vi "UHR-Fleezers Control (host) - 12.8.vi"() -> ()   [LabVIEW 2012] (continued)
        n423 = flat-sequence {
          tunnel: w684 -> [w688]
          tunnel: w685 -> [w689]
          tunnel: [w689] -> w681
          tunnel: [w688] -> w680
          tunnel: w681 -> [w694]
          tunnel: w680 -> [w693]
          tunnel: ["Cal @ (MHz)"] -> w678
          tunnel: [w698] -> w682
          tunnel: w678 -> [w698]
          tunnel: w682 -> [w707]
          tunnel: ["W/ Offset 1"] -> w679
          tunnel: w682 -> [w728]
          tunnel: w679 -> [w726]
          frame #0 {
            n424 = property on="Sample Channel\nFlow" class="Bool (strict)"("Val(Sgnl)"="Daq spot flow on") -> ()  [unwired: 2 in, 2 out]
            n425 = Wait (ms)(milliseconds to wait=u32 250) -> ()  [unwired: 1 out]
          }
          frame #1 {
            n426 = local read "Saved Stage Positions"() -> (w691:dbl[][])
            n427 = property on="Trap Delta (MHz)" class="DigNum (strict)"("Val(Sgnl)"="Cal @ (MHz)") -> ()  [unwired: 2 in, 2 out]
            n428 = local write "Stage Moving"(TRUE ("Stage Moving")) -> ()
            n429 = call "move to saved stage position.vi"("error in"=w693, "Stage VISA resource name in"=w694, "Position"="Cal Stage Position", "Saved Stage Positions"=w691) -> ("error out"=w692:errorcluster)  [unwired: 1 out]
            n430 = local write "Stage Control Serial Error"(w692) -> ()
          }
          frame #2 {
            n431 = local write "Stage Moving"(FALSE ("Stage Moving")) -> ()
            n432 = property on="Sample Channel\nFlow" class="Bool (strict)"("Val(Sgnl)"="Flow ON during cal?") -> ()  [unwired: 2 in, 2 out]
            n433 = call <vilib>:"Beep.vi"() -> ()  [unwired: 3 in, 9 out]
          }
          frame #3 {
            n434 = Wait (ms)(milliseconds to wait=u32 1000) -> ()  [unwired: 1 out]
          }
          frame #4 {
            n435 = property on="Save Calibration" class="Bool (strict)"("Val(Sgnl)"=TRUE ("Value (Signaling)")) -> ()  [unwired: 2 in, 2 out]
          }
          frame #5 {
            n436 = Wait (ms)(milliseconds to wait=u32 2000) -> ()  [unwired: 1 out]
          }
          frame #6 {
            # "Check to see if \nsaving done"
            n437 = while {
              stop <- w703 stop-if-true
              n438 = local read "Saving..."() -> (w704:bool)
              n439 = Wait (ms)(milliseconds to wait=u32 100) -> ()  [unwired: 1 out]
              n440 = Not(x=w704) -> (.not. x?=w703:bool)
            }
          }
          frame #7 {
            n441 = case shown="True" "W/ Offset 1" {
              tunnel: w707 -> [_ w708]
              frame False {
              }
              frame True {
                n442 = stacked-sequence {
                  tunnel: w708 -> [_ _ _ _ _ _ _ w725]
                  frame #0 {
                    n443 = property on="Trap Delta (MHz)" class="DigNum (strict)"("Val(Sgnl)"="Offset 1 Start (MHz)") -> ()  [unwired: 2 in, 2 out]
                    n444 = Replace Array Subset(array=u32[] [0] ("Index Values"), new element="Offset 1 Set", index=0) -> (w709:u32[])
                    n445 = property on="Saved AOD Raster Scan Parameter Sets" class="Arr (strict)"("Index Values"=w709) -> ()  [unwired: 2 in, 2 out]
                  }
                  frame #1 {
                    n446 = Wait (ms)(milliseconds to wait=u32 200) -> ()  [unwired: 1 out]
                  }
                  frame #2 {
                    n447 = property on="Load parameters" class="Bool (strict)"("Val(Sgnl)"=TRUE ("Value (Signaling)")) -> ()  [unwired: 2 in, 2 out]
                  }
                  frame #3 {
                    n448 = Wait (ms)(milliseconds to wait=u32 200) -> ()  [unwired: 1 out]
                  }
                  frame #4 {
                    n449 = property on="Trap Raster Scan" class="Bool (strict)"("Val(Sgnl)"=TRUE ("Value (Signaling)")) -> ()  [unwired: 2 in, 2 out]
                  }
                  frame #5 {
                    n450 = Wait (ms)(milliseconds to wait=u32 2000) -> ()  [unwired: 1 out]
                  }
                  frame #6 {
                    n451 = while {
                      stop <- w722 stop-if-true
                      n452 = local read "Raster Scanning..."() -> (w724:bool)
                      n453 = local read "Saving..."() -> (w720:bool)
                      n454 = Wait (ms)(milliseconds to wait=u32 100) -> ()  [unwired: 1 out]
                      n455 = Not(x=w720) -> (.not. x?=w719:bool)
                      n456 = Not(x=w724) -> (.not. x?=w721:bool)
                      n457 = And(x=w721, y=w719) -> (x .and. y?=w722:bool)
                    }
                  }
                  frame #7 {
                    n458 = property on="Trap Delta (MHz)" class="DigNum (strict)"("Val(Sgnl)"=w725) -> ()  [unwired: 2 in, 2 out]
                  }
                }
              }
            }
          }
          frame #8 {
            n459 = local read "Save ave N"() -> (w727:dbl)
            n460 = case shown="False" "W/ Offset 2" {
              tunnel: w728 -> [_ w735]
              tunnel: w727 -> [_ w734]
              tunnel: w726 -> [w730 _]
              frame False {
                n461 = case shown="False" w730 {
                  frame False {
                    n462 = Multiply(x="Cal read wait (s)", y=u32 1000 ("milliseconds to wait")) -> (x*y=w732:u32)
                    n463 = Wait (ms)(milliseconds to wait=w732) -> ()  [unwired: 1 out]
                  }
                  frame True {
                  }
                }
              }
              frame True {
                n464 = stacked-sequence {
                  tunnel: w735 -> [_ _ _ _ _ _ _ _ _ w756 _ _]
                  tunnel: w734 -> [_ _ _ _ _ _ _ _ _ w754 _ _]
                  frame #0 {
                    n465 = property on="Save ave N" class="DigNum (strict)"("Val(Sgnl)"=1.0 ("Value (Signaling)")) -> ()  [unwired: 2 in, 2 out]
                  }
                  frame #1 {
                    n466 = Wait (ms)(milliseconds to wait=u32 500) -> ()  [unwired: 1 out]
                  }
                  frame #2 {
                    n467 = property on="Trap Delta (MHz)" class="DigNum (strict)"("Val(Sgnl)"="Offset 2 Start (MHz)") -> ()  [unwired: 2 in, 2 out]
                    n468 = Replace Array Subset(array=u32[] [0] ("Index Values"), new element="Offset 2 Set", index=0) -> (w740:u32[])
                    n469 = property on="Saved AOD Raster Scan Parameter Sets" class="Arr (strict)"("Index Values"=w740) -> ()  [unwired: 2 in, 2 out]
                  }
                  frame #3 {
                    n470 = Wait (ms)(milliseconds to wait=u32 500) -> ()  [unwired: 1 out]
                  }
                  frame #4 {
                    n471 = property on="Load parameters" class="Bool (strict)"("Val(Sgnl)"=TRUE ("Value (Signaling)")) -> ()  [unwired: 2 in, 2 out]
                  }
                  frame #5 {
                    n472 = Wait (ms)(milliseconds to wait=u32 500) -> ()  [unwired: 1 out]
                  }
                  frame #6 {
                    n473 = property on="Trap Raster Scan" class="Bool (strict)"("Val(Sgnl)"=TRUE ("Value (Signaling)")) -> ()  [unwired: 2 in, 2 out]
                  }
                  frame #7 {
                    n474 = Wait (ms)(milliseconds to wait=u32 2000) -> ()  [unwired: 1 out]
                  }
                  frame #8 {
                    n475 = while {
                      stop <- w749 stop-if-true
                      n476 = local read "Raster Scanning..."() -> (w752:bool)
                      n477 = local read "Saving..."() -> (w750:bool)
                      n478 = Wait (ms)(milliseconds to wait=u32 100) -> ()  [unwired: 1 out]
                      n479 = Not(x=w750) -> (.not. x?=w748:bool)
                      n480 = Not(x=w752) -> (.not. x?=w751:bool)
                      n481 = And(x=w751, y=w748) -> (x .and. y?=w749:bool)
                    }
                  }
                  frame #9 {
                    n482 = property on="Trap Delta (MHz)" class="DigNum (strict)"("Val(Sgnl)"=w756) -> ()  [unwired: 2 in, 2 out]
                    n483 = property on="Saved AOD Raster Scan Parameter Sets" class="Arr (strict)"("Index Values"=u32[] [0]) -> ()  [unwired: 2 in, 2 out]
                    n484 = property on="Save ave N" class="DigNum (strict)"("Val(Sgnl)"=w754) -> ()  [unwired: 2 in, 2 out]
                  }
                  frame #10 {
                    n485 = Wait (ms)(milliseconds to wait=u32 500) -> ()  [unwired: 1 out]
                  }
                  frame #11 {
                    n486 = property on="Load parameters" class="Bool (strict)"("Val(Sgnl)"=TRUE ("Value (Signaling)")) -> ()  [unwired: 2 in, 2 out]
                  }
                }
              }
            }
          }
          frame #9 {
            n487 = property on="Read Cal" class="Bool (strict)"("Val(Sgnl)"=TRUE ("Value (Signaling)")) -> ()  [unwired: 2 in, 2 out]
          }
          frame #10 {
            n488 = Wait (ms)(milliseconds to wait=u32 1000) -> ()  [unwired: 1 out]
          }
          frame #11 {
            n489 = property on="Fish for Tether" class="Bool (strict)"("Val(Sgnl)"=TRUE ("Value (Signaling)")) -> ()  [unwired: 2 in, 2 out]
          }
        }
        n490 = local write "Cal/Data Acq. Spot"(FALSE ("Cal/Data Acq. Spot")) -> ()
      }
      event "Dump Beads": Value Change {
        n491 = event-data() -> ()  [unwired: 1 in, 5 out]
        n492 = flat-sequence {
          tunnel: ["Dump spot flow on?"] -> w762
          tunnel: [w773] -> w763
          tunnel: w762 -> [w773]
          tunnel: w766 -> [w778]
          tunnel: w765 -> [w777]
          tunnel: [w775] -> w764
          tunnel: w763 -> [w775]
          tunnel: w764 -> [w788]
          frame #0 {
            w767 = FALSE ("Value (Signaling)")
            n493 = local read "Saving..."() -> (w769:bool)
            n494 = local write "Dump Beads"(FALSE ("Dump Beads")) -> ()
            n495 = property on="Inject Pump 3" class="Bool (strict)"("Val(Sgnl)"=w767) -> ()  [unwired: 2 in, 2 out]
            n496 = property on="Inject Pump 1" class="Bool (strict)"("Val(Sgnl)"=w767) -> ()  [unwired: 2 in, 2 out]
            n497 = local write "Stop Saving"(w769) -> ()
          }
          frame #1 {
            w770 = FALSE ("Fl. Triggered...")
            n498 = case shown="True" "Dump spot flow on?" {
              frame False {
              }
              frame True {
                n499 = property on="Sample Channel\nFlow" class="Bool (strict)"("Val(Sgnl)"=TRUE ("Stage Moving")) -> ()  [unwired: 2 in, 2 out]
              }
            }
            n500 = local write "Fl. Triggered..."(w770) -> ()
            n501 = local write "Tether"(w770) -> ()
            n502 = property on="Green Laser ON" class="Bool (strict)"("Val(Sgnl)"=w770) -> ()  [unwired: 2 in, 2 out]
            n503 = property on="Trap Pos. FB ON" class="Bool (strict)"("Val(Sgnl)"=w770) -> ()  [unwired: 2 in, 2 out]
            n504 = property on="Trap Trig. Fl." class="Bool (strict)"("Val(Sgnl)"=w770) -> ()  [unwired: 2 in, 2 out]
            n505 = property on="Fl. Triggered..." class="Bool (strict)"("Val(Sgnl)"=w770) -> ()  [unwired: 2 in, 2 out]
            n506 = property on="Dip for Protein" class="Bool (strict)"("Val(Sgnl)"=w770) -> ()  [unwired: 2 in, 2 out]
            n507 = property on="Pause dwell" class="Bool (strict)"("Val(Sgnl)"=w770) -> ()  [unwired: 2 in, 2 out]
          }
          frame #2 {
            n508 = property on="Trap Pos. FB Offset Factor" class="DigNum (strict)"("Val(Sgnl)"=i64 0 ("Value (Signaling)")) -> ()  [unwired: 2 in, 2 out]
          }
          frame #3 {
            n509 = local read "Saved Stage Positions"() -> (w779:dbl[][])
            n510 = local write "Stage Moving"(TRUE ("Stage Moving")) -> ()
            n511 = Array Subset(array=w779, index (row)=3 ("index"), length (row)=1 ("length"), index (col)=1 ("index"), length (col)=3 ("length")) -> (w784:dbl[][])
            n512 = Reshape Array(w784, 3 ("dimension size")) -> (w782:dbl[])
            n513 = Array To Cluster(array=w782) -> (cluster=w781:cluster{"[0]":dbl, "[1]":dbl, "[2]":dbl})
            n514 = call "Set Stage Position.vi"("Position"=w781, "error in"=w777, "VISA resource name in"=w778) -> ()  [unwired: 3 out]
          }
          frame #4 {
            w789 = FALSE ("Value (Signaling)")
            n515 = case shown="True" w788 {
              frame False {
              }
              frame True {
                n516 = property on="Sample Channel\nFlow" class="Bool (strict)"("Val(Sgnl)"=FALSE ("Stage Moving")) -> ()  [unwired: 2 in, 2 out]
              }
            }
            n517 = property on="Trap 1 (ON/OFF)" class="Bool (strict)"("Val(Sgnl)"=w789) -> ()  [unwired: 2 in, 2 out]
            n518 = property on="Trap 2 (ON/OFF)" class="Bool (strict)"("Val(Sgnl)"=w789) -> ()  [unwired: 2 in, 2 out]
            n519 = call <vilib>:"Beep.vi"() -> ()  [unwired: 3 in, 9 out]
          }
          frame #5 {
            n520 = property on="Move Cap. 2 (ADig Top)" class="Bool (strict)"("Val(Sgnl)"=TRUE ("Value (Signaling)")) -> ()  [unwired: 2 in, 2 out]
            n521 = property on="Tab Control" class="TabCtl (strict)"("Val(Sgnl)"=T26."Status" ("Value (Signaling)")) -> ()  [unwired: 2 in, 2 out]
          }
        }
      }
      event "Dip for Protein": Value Change {
        n522 = event-data() -> ()  [unwired: 1 in, 5 out]
        n523 = case shown="True" "Dip for Protein" {
          tunnel: w795 -> [_ w797]
          tunnel: w794 -> [_ w796]
          frame False {
          }
          frame True {
            n524 = while {
              tunnel: w797 -> [w808]
              tunnel: w796 -> [w807]
              i -> [w802]
              stop <- w804 stop-if-true
              n525 = Increment(x=w802) -> (x+1=→"Dip #":i32)
              n526 = flat-sequence {
                tunnel: w807 -> [w819]
                tunnel: w808 -> [w820]
                tunnel: [w820] -> w812
                tunnel: [w819] -> w811
                tunnel: [w813] -> w798
                tunnel: [w825] -> w806
                tunnel: [w826] -> w805
                tunnel: w812 -> [w827]
                tunnel: w811 -> [w828]
                tunnel: [w823] -> w799
                tunnel: w798 -> [w823]
                tunnel: [w836] -> w810
                tunnel: w806 -> [w836]
                tunnel: [w835] -> w809
                tunnel: w805 -> [w835]
                tunnel: [w832] -> w803
                tunnel: [w831] -> w800
                tunnel: w799 -> [w831]
                tunnel: w809 -> [w856]
                tunnel: w810 -> [w857]
                tunnel: w803 -> [w858]
                tunnel: w800 -> [w855]
                tunnel: [w914] -> w804
                frame #0 {
                  n527 = local read "Trap Pos. FB ON"() -> (w813:bool)
                  n528 = Compound Arithmetic op=AND("Flow ON\nduring dip?", "FB OFF when \nflow ON", w813) -> (w814:bool)
                  n529 = case shown="True" "Move trap \nbefore dip move?" {
                    frame False {
                    }
                    frame True {
                      n530 = property on="Trap Delta (MHz)" class="DigNum (strict)"("Val(Sgnl)"="Dipping Delta (MHz)") -> ()  [unwired: 2 in, 2 out]
                    }
                  }
                  n531 = property on="Green Laser ON" class="Bool (strict)"("Val(Sgnl)"="Green ON\nbefore dip?") -> ()  [unwired: 2 in, 2 out]
                  n532 = property on="Sample Channel\nFlow" class="Bool (strict)"("Val(Sgnl)"="Flow ON\nduring dip?") -> ()  [unwired: 2 in, 2 out]
                  n533 = case shown="True" w814 {
                    frame False {
                    }
                    frame True {
                      n534 = property on="Trap Pos. FB ON" class="Bool (strict)"("Val(Sgnl)"=FALSE ("Value (Signaling)")) -> ()  [unwired: 2 in, 2 out]
                    }
                  }
                }
                frame #1 {
                  n535 = local read "Saved Stage Positions"() -> (w830:dbl[][])
                  n536 = local write "Cancel dwell"(FALSE ("Cancel dwell")) -> ()
                  n537 = call "move to saved stage position.vi"("error in"=w828, "Stage VISA resource name in"=w827, "Position"="Dip Stage \nPosition", "Saved Stage Positions"=w830) -> ("VISA resource name out"=w825:refnum<visa-resource-name>, "error out"=w826:errorcluster)
                }
                frame #2 {
                  n538 = node-c288() -> (w834:T23)  [unwired: 4 in]
                  n539 = timed-loop {
                    timing: w834 -> [_]
                    timing-out: [_] -> w833
                    tunnel: [w840] -> w832
                    i -> [w837]
                    stop <- w841 stop-if-true
                    n540 = node-c288() -> ()  [unwired: 1 in, 1 out]
                    n541 = Greater Or Equal?(x=w837, y="Dip Duration (s)") -> (x >= y?=w849:bool)
                    n542 = local read "Dip for Protein"() -> (w842:bool)
                    n543 = local read "Dump Beads"() -> (w839:bool)
                    n544 = local read "Cancel dwell"() -> (w848:bool)
                    n545 = local read "Pause dwell"() -> (w845:bool)
                    n546 = Not(x=w842) -> (.not. x?=w847:bool)
                    n547 = Compound Arithmetic op=OR(w848, w849, w847) -> (w846:bool)
                    n548 = Select(t=FALSE, s=w845, f=w846) -> (s? t:f=w843:bool)
                    n549 = Not(x=w839) -> (.not. x?=w838:bool)
                    n550 = node-c288() -> ()  [unwired: 1 in, 1 out]
                    n551 = And(x=w842, y=w838) -> (x .and. y?=w840:bool)
                    n552 = Or(x=w843, y=w839) -> (x .or. y?=w841:bool)
                    "Dip Time (s)" <- w837
                  }
                  n553 = node-c288(w833) -> ()  [unwired: 1 out]
                }
                frame #3 {
                  n554 = case shown="True" w858 {
                    tunnel: w857 -> [_ w863]
                    tunnel: w856 -> [_ w862]
                    tunnel: w855 -> [_ w859]
                    frame False {
                    }
                    frame True {
                      n555 = flat-sequence {
                        tunnel: w862 -> [w867]
                        tunnel: w863 -> [w868]
                        tunnel: [w868] -> w861
                        tunnel: [w867] -> w860
                        tunnel: w859 -> [w864]
                        tunnel: w861 -> [w878]
                        tunnel: w860 -> [w877]
                        tunnel: w859 -> [w886]
                        frame #0 {
                          n556 = local read "Sample Channel\nFlow"() -> (w866:bool)
                          n557 = case shown="True" w866 {
                            tunnel: "Flow ON \nduring return\nfrom dip?" -> [w869 w872]
                            tunnel: w864 -> [_ w871]
                            frame False {
                              n558 = case shown="True" w869 {
                                frame False {
                                }
                                frame True {
                                n559 = property on="Sample Channel\nFlow" class="Bool (strict)"("Val(Sgnl)"=TRUE ("Value (Signaling)")) -> ()  [unwired: 2 in, 2 out]
                                }
                              }
                            }
                            frame True {
                              n560 = case shown="False" w872 {
                                tunnel: w871 -> [w873 _]
                                frame False {
                                n561 = property on="Trap Pos. FB ON" class="Bool (strict)"("Val(Sgnl)"=w873) -> ()  [unwired: 2 in, 2 out]
                                n562 = property on="Sample Channel\nFlow" class="Bool (strict)"("Val(Sgnl)"=FALSE ("Value (Signaling)")) -> ()  [unwired: 2 in, 2 out]
                                }
                                frame True {
                                }
                              }
                            }
                          }
                        }
                        frame #1 {
                          # "For turning on green laser before stage reaches lower spot"
                          n563 = case shown="True" "Green ON\nafter start\nreturn?" {
                            frame False {
                            }
                            frame True {
                              n564 = flat-sequence {
                                frame #0 {
                                n565 = Multiply(x="Green delay after \nstart return (s)", y=1000.0) -> (x*y=w883:dbl)
                                n566 = Wait (ms)(milliseconds to wait=w883) -> ()  [unwired: 1 out]
                                }
                                frame #1 {
                                n567 = property on="Green Laser ON" class="Bool (strict)"("Val(Sgnl)"=TRUE ("Value (Signaling)")) -> ()  [unwired: 2 in, 2 out]
                                }
                              }
                            }
                          }
                          n568 = local read "Saved Stage Positions"() -> (w881:dbl[][])
                          n569 = local write "Cancel dwell"(FALSE ("Cancel dwell")) -> ()
                          n570 = call "move to saved stage position.vi"("error in"=w877, "Stage VISA resource name in"=w878, "Position"="Return Stage \nPosition", "Saved Stage Positions"=w881) -> ("error out"=w879:errorcluster)  [unwired: 1 out]
                          n571 = local write "Stage Control Serial Error"(w879) -> ()
                        }
                        frame #2 {
                          n572 = property on="Trap Pos. FB ON" class="Bool (strict)"("Val(Sgnl)"=w886) -> ()  [unwired: 2 in, 2 out]
                          n573 = case shown="True" "Green ON \nafter return?" {
                            frame False {
                            }
                            frame True {
                              n574 = property on="Green Laser ON" class="Bool (strict)"("Val(Sgnl)"=TRUE ("Value (Signaling)")) -> ()  [unwired: 2 in, 2 out]
                            }
                          }
                          n575 = case shown="True" "Move trap after return?" {
                            frame False {
                            }
                            frame True {
                              n576 = property on="Trap Delta (MHz)" class="DigNum (strict)"("Val(Sgnl)"="Dip Trap Delta 2 (MHz)") -> ()  [unwired: 2 in, 2 out]
                            }
                          }
                          n577 = case shown="True" "Save data after return?" {
                            frame False {
                            }
                            frame True {
                              n578 = property on="Start Saving" class="Bool (strict)"("Val(Sgnl)"=TRUE ("Value (Signaling)")) -> ()  [unwired: 2 in, 2 out]
                            }
                          }
                          n579 = property on="Sample Channel\nFlow" class="Bool (strict)"("Val(Sgnl)"="Flow ON\nduring daq?") -> ()  [unwired: 2 in, 2 out]
                        }
                        frame #3 {
                          n580 = node-c288() -> (w895:T23)  [unwired: 4 in]
                          n581 = timed-loop {
                            timing: w895 -> [_]
                            timing-out: [_] -> w894
                            i -> [w896]
                            stop <- w898 stop-if-true
                            n582 = node-c288() -> ()  [unwired: 1 in, 1 out]
                            n583 = local read "Dump Beads"() -> (w897:bool)
                            n584 = Greater Or Equal?(x=w896, y="Dwell Duration (s)") -> (x >= y?=w903:bool)
                            n585 = local read "Dip for Protein"() -> (w900:bool)
                            n586 = Not(x=w900) -> (.not. x?=w899:bool)
                            n587 = Compound Arithmetic op=OR(w903, "Cancel dwell", w899) -> (w902:bool)
                            n588 = node-c288() -> ()  [unwired: 1 in, 1 out]
                            n589 = Select(t=FALSE, s="Pause dwell", f=w902) -> (s? t:f=w905:bool)
                            n590 = Or(x=w905, y=w897) -> (x .or. y?=w898:bool)
                            "Dwell Time (s)" <- w896
                          }
                          n591 = node-c288(w894) -> ()  [unwired: 1 out]
                        }
                      }
                    }
                  }
                }
                frame #4 {
                  n592 = local read "Dip for Protein"() -> (w915:bool)
                  n593 = local read "Dump Beads"() -> (w912:bool)
                  n594 = local write "Cancel dwell"(FALSE ("Cancel dwell")) -> ()
                  n595 = Not(x=w915) -> (.not. x?=w916:bool)
                  n596 = Not(x="Cont. Repeat Dipping?") -> (.not. x?=w918:bool)
                  n597 = Compound Arithmetic op=OR(w916, w918, w912) -> (w914:bool)
                }
              }
            }
          }
        }
      }
      event "Profile": Value Change {
        n598 = event-data() -> ()  [unwired: 1 in, 5 out]
        n599 = flat-sequence {
          tunnel: w927 -> [w930]
          tunnel: w926 -> [w938]
          tunnel: [w932] -> w925
          tunnel: [w931] -> w924
          tunnel: [w929] -> w922
          tunnel: [w928] -> w919
          tunnel: w925 -> [w945]
          tunnel: w924 -> [w944]
          tunnel: [w942] -> w923
          tunnel: w922 -> [w943]
          tunnel: [w941] -> w921
          tunnel: [w940] -> w920
          tunnel: w919 -> [w940]
          tunnel: w923 -> [w949]
          tunnel: w921 -> [w948]
          tunnel: w920 -> [w947]
          frame #0 {
            n600 = call "Read Stage Position.vi"("error in"=w938, "VISA resource name in"=w930) -> ("Current Position"=w928:cluster{dbl, dbl, dbl}, "error out"=w931:errorcluster, "VISA resource name out"=w929:refnum<visa-resource-name>)  [unwired: 1 out]
            "Current Position" <- w928
            n601 = local write "Stage Control Serial Error"(w931) -> ()
            n602 = Unbundle(w928) -> (w935:dbl, w937:dbl, w933:dbl)
            n603 = Add(x=w937, y="Y change (mm)") -> (x+y=w934:dbl)
            n604 = Bundle(w935, w934, w933) -> (w932:cluster{dbl, dbl, dbl})  [unwired: 1 in]
          }
          frame #1 {
            # "move to new position and start saving"
            n605 = local write "Stage Moving"(TRUE ("Stage Moving")) -> ()
            n606 = local write "Start Saving"(TRUE ("Start Saving")) -> ()
            n607 = call "Set Stage Position.vi"("Position"=w945, "error in"=w944, "VISA resource name in"=w943) -> ("error out"=w941:errorcluster, "VISA resource name out"=w942:refnum<visa-resource-name>)  [unwired: 1 out]
          }
          frame #2 {
            # "go back to start"
            n608 = call "Set Stage Position.vi"("Position"=w947, "error in"=w948, "VISA resource name in"=w949) -> ()  [unwired: 3 out]
          }
          frame #3 {
            # "stop saving"
            n609 = local write "Stop Saving"(TRUE ("Stop Saving")) -> ()
            n610 = local write "Stage Moving"(FALSE ("Stage Moving")) -> ()
          }
        }
      }
      event "Move to Position 1", "Move to Position 2", "Move to Position 3", "Move to Position 4", "Move to Position 5", "Lower Ch. Cap.": Value Change {
        n611 = event-data() -> ()  [unwired: 1 in, 5 out]
        n612 = Or(x="Move to Position 5", y="Lower Ch. Cap.") -> (x .or. y?=w955:bool)
        n613 = Build Array("Move to Position 1", "Move to Position 2", "Move to Position 3", "Move to Position 4", w955) -> (w958:bool[])
        n614 = Boolean Array To Number(Boolean array=w958) -> (number=w957:u32)
        n615 = Logarithm Base 2(1:w957) -> (0:w956:dbl)
        n616 = flat-sequence {
          tunnel: w956 -> [w967]
          tunnel: w953 -> [w965]
          tunnel: w952 -> [w964]
          frame #0 {
            n617 = local read "Saved Stage Positions"() -> (w975:dbl[][])
            n618 = Array Subset(array=w975, index (row)=w967, length (row)=1 ("length"), index (col)=1 ("index"), length (col)=3 ("length")) -> (w972:dbl[][])
            n619 = Reshape Array(w972, 3 ("dimension size")) -> (w970:dbl[])
            n620 = Array To Cluster(array=w970) -> (cluster=w969:cluster{"[0]":dbl, "[1]":dbl, "[2]":dbl})
            n621 = call "Set Stage Position.vi"("Position"=w969, "error in"=w964, "VISA resource name in"=w965) -> ("error out"=w968:errorcluster)  [unwired: 2 out]
            n622 = local write "Stage Moving"(TRUE ("Stage Moving")) -> ()
            n623 = local write "Stage Control Serial Error"(w968) -> ()
          }
          frame #1 {
            n624 = local write "Stage Moving"(FALSE ("Stage Moving")) -> ()
            n625 = call <vilib>:"Beep.vi"() -> ()  [unwired: 3 in, 9 out]
          }
        }
      }
      event "Got ADig bead": Value Change {
        n626 = event-data() -> ()  [unwired: 1 in, 5 out]
        n627 = flat-sequence {
          frame #0 {
            n628 = local read "Cap 1 Samp Flow ON"() -> (w979:bool)
            n629 = case shown="True" w979 {
              frame False {
              }
              frame True {
                n630 = property on="Sample Channel\nFlow" class="Bool (strict)"("Val(Sgnl)"=TRUE ("Value (Signaling)")) -> ()  [unwired: 2 in, 2 out]
              }
            }
          }
          frame #1 {
            n631 = property on="Inject Pump 3" class="Bool (strict)"("Val(Sgnl)"=FALSE ("Value (Signaling)")) -> ()  [unwired: 2 in, 2 out]
          }
          frame #2 {
            n632 = property on="Move Cap. 1 (DNA Bottom)" class="Bool (strict)"("Val(Sgnl)"=TRUE ("Value (Signaling)")) -> ()  [unwired: 2 in, 2 out]
          }
        }
      }
      event "Force FB Data\nScript": Value Change {
        n633 = event-data() -> ()  [unwired: 1 in, 5 out]
        n634 = flat-sequence {
          tunnel: w988 -> [w992]
          tunnel: w989 -> [w993]
          tunnel: [w993] -> w984
          tunnel: [w992] -> w983
          tunnel: w984 -> [w996]
          tunnel: w983 -> [w995]
          tunnel: ["Trap Trig Fl."] -> w985
          tunnel: [w1021] -> w986
          tunnel: w985 -> [w1021]
          tunnel: [w1025] -> w987
          tunnel: w986 -> [w1025]
          tunnel: w987 -> [w1027]
          frame #0 {
            n635 = property on="Trap Delta (MHz)" class="DigNum (strict)"("Val(Sgnl)"="Trap Delta Before Moving") -> ()  [unwired: 2 in, 2 out]
          }
          frame #1 {
            n636 = local read "Saved Stage Positions"() -> (w998:dbl[][])
            n637 = local write "FB Trap Pos Offset"(0.0 ("FB Trap Pos Offset")) -> ()
            n638 = property on="Trap Pos. FB Offset Factor" class="DigNum (strict)"("Val(Sgnl)"=i64 0 ("Value (Signaling)")) -> ()  [unwired: 2 in, 2 out]
            n639 = local write "Stage Moving"(TRUE ("Stage Moving")) -> ()
            n640 = call "move to saved stage position.vi"("error in"=w995, "Stage VISA resource name in"=w996, "Position"="Stage Position To Establish FB", "Saved Stage Positions"=w998) -> ("error out"=w994:errorcluster)  [unwired: 1 out]
            n641 = local write "Stage Control Serial Error"(w994) -> ()
          }
          frame #2 {
            n642 = call <vilib>:"Beep.vi"() -> ()  [unwired: 3 in, 9 out]
            n643 = Multiply(x="Wait (s)", y=u32 1000 ("milliseconds to wait")) -> (x*y=w1005:u32)
            n644 = property on="Trap Delta (MHz)" class="DigNum (strict)"("Val(Sgnl)"="Starting \nTrap Delta (MHz)") -> ()  [unwired: 2 in, 2 out]
            n645 = local write "Stage Moving"(FALSE ("Stage Moving")) -> ()
            n646 = Wait (ms)(milliseconds to wait=w1005) -> ()  [unwired: 1 out]
            n647 = property on="Tab Control 2" class="TabCtl (strict)"("Val(Sgnl)"=T6."Feedback on Trap Position" ("Value (Signaling)")) -> ()  [unwired: 2 in, 2 out]
            n648 = property on="Tab Control" class="TabCtl (strict)"("Val(Sgnl)"=T27."Trap Control (RF)" ("Value (Signaling)")) -> ()  [unwired: 2 in, 2 out]
          }
          frame #3 {
            n649 = property on="Set Reading to\nSetpoint" class="Bool (strict)"("Val(Sgnl)"=TRUE ("Value (Signaling)")) -> ()  [unwired: 2 in, 2 out]
            n650 = Wait (ms)(milliseconds to wait=u32 500) -> ()  [unwired: 1 out]
          }
          frame #4 {
            n651 = property on="Trap Pos. FB ON" class="Bool (strict)"("Val(Sgnl)"=TRUE ("Value (Signaling)")) -> ()  [unwired: 2 in, 2 out]
            n652 = Wait (ms)(milliseconds to wait=u32 250) -> ()  [unwired: 1 out]
          }
          frame #5 {
            n653 = case shown="False" "Trap Trig Fl." {
              frame False {
                n654 = case shown="True" "Green ON after FB ON?" {
                  selector: "Green ON after FB ON?" -> [_ w1020]
                  frame False {
                  }
                  frame True {
                    n655 = property on="Green Laser ON" class="Bool (strict)"("Val(Sgnl)"=w1020) -> ()  [unwired: 2 in, 2 out]
                  }
                }
              }
              frame True {
              }
            }
            n656 = case shown="True" "Remove Action Offset" {
              tunnel: TRUE ("Value (Signaling)") -> [w1017 w1018]
              frame False {
                n657 = property on="Remove Unwinding Offset" class="Bool (strict)"("Val(Sgnl)"=w1017) -> ()  [unwired: 2 in, 2 out]
              }
              frame True {
                n658 = property on="Remove Action Offset" class="Bool (strict)"("Val(Sgnl)"=w1018) -> ()  [unwired: 2 in, 2 out]
              }
            }
            n659 = Wait (ms)(milliseconds to wait=u32 250) -> ()  [unwired: 1 out]
          }
          frame #6 {
            n660 = property on="Start Saving" class="Bool (strict)"("Val(Sgnl)"=TRUE ("Value (Signaling)")) -> ()  [unwired: 2 in, 2 out]
            n661 = Wait (ms)(milliseconds to wait=u32 5000) -> ()  [unwired: 1 out]
          }
          frame #7 {
            w1024 = TRUE ("Value (Signaling)")
            n662 = property on="Rem fb disp offset" class="Bool (strict)"("Val(Sgnl)"=w1024) -> ()  [unwired: 2 in, 2 out]
            n663 = property on="Remove Offset" class="Bool (strict)"("Val(Sgnl)"=w1024) -> ()  [unwired: 2 in, 2 out]
            n664 = Wait (ms)(milliseconds to wait=u32 100) -> ()  [unwired: 1 out]
          }
          frame #8 {
            n665 = case shown="True" w1027 {
              frame False {
              }
              frame True {
                n666 = local write "Trap Trig. Fl."(TRUE ("Value (Signaling)")) -> ()
              }
            }
          }
          frame #9 {
            n667 = case shown="True" "Start dipping after?" {
              frame False {
              }
              frame True {
                n668 = flat-sequence {
                  frame #0 {
                    n669 = Multiply(x="Delay before dipping (s)", y=1000.0) -> (x*y=w1031:dbl)
                    n670 = Wait (ms)(milliseconds to wait=w1031) -> ()  [unwired: 1 out]
                  }
                  frame #1 {
                    n671 = property on="Dip for Protein" class="Bool (strict)"("Val(Sgnl)"=TRUE ("Value (Signaling)")) -> ()  [unwired: 2 in, 2 out]
                    n672 = local write "Scripts"(T1."Dipping" ("Scripts")) -> ()
                  }
                }
              }
            }
          }
        }
      }
      event "Fixed Traps Data\nScript": Value Change {
        n673 = event-data() -> ()  [unwired: 1 in, 5 out]
        n674 = flat-sequence {
          frame #0 {
            n675 = case shown="True" "Green ON" {
              frame False {
              }
              frame True {
                n676 = property on="Green Laser ON" class="Bool (strict)"("Val(Sgnl)"=TRUE) -> ()  [unwired: 2 in, 2 out]
              }
            }
            n677 = local write "Offset (nm)"(0.0 ("Offset (nm)")) -> ()
            n678 = property on="Sample Channel\nFlow" class="Bool (strict)"("Val(Sgnl)"=FALSE ("Value (Signaling)")) -> ()  [unwired: 2 in, 2 out]
            n679 = property on="Trap Delta (MHz)" class="DigNum (strict)"("Val(Sgnl)"="Fixed Traps Trap Delta (MHz)") -> ()  [unwired: 2 in, 2 out]
          }
          frame #1 {
            n680 = Wait (ms)(milliseconds to wait=u32 1000) -> ()  [unwired: 1 out]
          }
          frame #2 {
            n681 = local write "Start Saving"(TRUE ("Start Saving")) -> ()
          }
          frame #3 {
            n682 = local read "Bead Sep. Int. Time (s)"() -> (w1042:dbl)
            n683 = Multiply(x=w1042, y=1000.0) -> (x*y=w1044:dbl)
            n684 = Wait (ms)(milliseconds to wait=w1044) -> ()  [unwired: 1 out]
          }
          frame #4 {
            n685 = property on="Remove Offset" class="Bool (strict)"("Val(Sgnl)"=TRUE ("Value (Signaling)")) -> ()  [unwired: 2 in, 2 out]
          }
          frame #5 {
            n686 = property on="Dip for Protein" class="Bool (strict)"("Val(Sgnl)"="Start dipping after?") -> ()  [unwired: 2 in, 2 out]
          }
        }
      }
      event "Got DNA bead": Value Change {
        n687 = event-data() -> ()  [unwired: 1 in, 5 out]
        n688 = flat-sequence {
          frame #0 {
            n689 = local read "Daq spot flow on"() -> (w1049:bool)
            n690 = case shown="True" w1049 {
              frame False {
              }
              frame True {
                n691 = property on="Sample Channel\nFlow" class="Bool (strict)"("Val(Sgnl)"=TRUE ("Value (Signaling)")) -> ()  [unwired: 2 in, 2 out]
              }
            }
            n692 = property on="Got DNA bead" class="Bool"("Key Focus"=FALSE) -> ()  [unwired: 2 in, 2 out]
          }
          frame #1 {
            n693 = property on="Inject Pump 1" class="Bool (strict)"("Val(Sgnl)"=FALSE ("Value (Signaling)")) -> ()  [unwired: 2 in, 2 out]
          }
          frame #2 {
            n694 = property on="Cal/Data Acq. Spot" class="Bool (strict)"("Val(Sgnl)"=TRUE ("Value (Signaling)")) -> ()  [unwired: 2 in, 2 out]
          }
        }
      }
      event "Take Stepping Data": Value Change {
        n695 = event-data() -> ()  [unwired: 1 in, 5 out]
        n696 = local read "Save ave N"() -> (w1061:dbl)
        n697 = flat-sequence {
          tunnel: w1061 -> [w1063]
          tunnel: [w1063] -> w1056
          tunnel: [w1065] -> w1057
          tunnel: w1056 -> [w1065]
          tunnel: [w1067] -> w1058
          tunnel: w1057 -> [w1067]
          tunnel: [w1070] -> w1059
          tunnel: w1058 -> [w1070]
          tunnel: [w1072] -> w1060
          tunnel: w1059 -> [w1072]
          tunnel: [w1074] -> w1054
          tunnel: w1060 -> [w1074]
          tunnel: w1054 -> [w1077]
          tunnel: [w1077] -> w1053
          tunnel: w1053 -> [w1078]
          tunnel: [w1078] -> w1055
          tunnel: w1055 -> [w1084]
          frame #0 {
            n698 = property on="Save ave N" class="DigNum (strict)"("Val(Sgnl)"="Save ave factor") -> ()  [unwired: 2 in, 2 out]
          }
          frame #1 {
            n699 = Wait (ms)(milliseconds to wait=u32 100) -> ()  [unwired: 1 out]
          }
          frame #2 {
            n700 = local read "Offset 2 Start (MHz)"() -> (w1069:dbl)
            n701 = property on="Saved AOD Raster Scan Parameter Sets" class="Arr (strict)"("Index Values"=u32[] [2]) -> ()  [unwired: 2 in, 2 out]
            n702 = property on="Trap Delta (MHz)" class="DigNum (strict)"("Val(Sgnl)"=w1069) -> ()  [unwired: 2 in, 2 out]
          }
          frame #3 {
            n703 = property on="Load parameters" class="Bool (strict)"("Val(Sgnl)"=TRUE ("Value (Signaling)")) -> ()  [unwired: 2 in, 2 out]
          }
          frame #4 {
            n704 = Wait (ms)(milliseconds to wait=u32 100) -> ()  [unwired: 1 out]
          }
          frame #5 {
            n705 = property on="Trap Raster Scan" class="Bool (strict)"("Val(Sgnl)"=TRUE ("Value (Signaling)")) -> ()  [unwired: 2 in, 2 out]
          }
          frame #6 {
            n706 = Wait (ms)(milliseconds to wait=u32 1000) -> ()  [unwired: 1 out]
          }
          frame #7 {
            n707 = while {
              stop <- w1081 stop-if-true
              n708 = local read "Raster Scanning..."() -> (w1083:bool)
              n709 = local read "Saving..."() -> (w1082:bool)
              n710 = Not(x=w1082) -> (.not. x?=w1079:bool)
              n711 = Not(x=w1083) -> (.not. x?=w1080:bool)
              n712 = And(x=w1080, y=w1079) -> (x .and. y?=w1081:bool)
            }
          }
          frame #8 {
            n713 = property on="Save ave N" class="DigNum (strict)"("Val(Sgnl)"=w1084) -> ()  [unwired: 2 in, 2 out]
          }
        }
      }
      event "Step Size (nm)": Value Change {
        n714 = event-data() -> ()  [unwired: 1 in, 5 out]
        n715 = flat-sequence {
          frame #0 {
            n716 = property on="Saved AOD Raster Scan Parameter Sets" class="Arr (strict)"("Index Values"=u32[] [1]) -> ()  [unwired: 2 in, 2 out]
          }
          frame #1 {
            n717 = Multiply(x="N Steps", y="Step Size (nm)") -> (x*y=w1086:dbl)
            n718 = property on="Scan Speed AOD (nm/s) 2" class="DigNum (strict)"("Value"="Step Size (nm)") -> ()  [unwired: 2 in, 2 out]
            n719 = property on="Step Size AOD (nm) 2" class="DigNum (strict)"("Value"="Step Size (nm)") -> ()  [unwired: 2 in, 2 out]
            n720 = property on="Scan Range AOD (nm) 2" class="DigNum (strict)"("Value"=w1086) -> ()  [unwired: 2 in, 2 out]
          }
        }
      }
      event "Take Detection Laser\nImage": Value Change {
        n721 = event-data() -> ()  [unwired: 1 in, 5 out]
        n722 = flat-sequence {
          tunnel: [w1114] -> w1104
          tunnel: [w1113] -> w1097
          tunnel: [w1112] -> w1089
          tunnel: [w1117] -> w1105
          tunnel: w1104 -> [w1117]
          tunnel: [w1116] -> w1098
          tunnel: w1097 -> [w1116]
          tunnel: [w1115] -> w1090
          tunnel: w1089 -> [w1115]
          tunnel: [w1121] -> w1106
          tunnel: w1105 -> [w1121]
          tunnel: [w1120] -> w1099
          tunnel: w1098 -> [w1120]
          tunnel: [w1119] -> w1091
          tunnel: w1090 -> [w1119]
          tunnel: [w1127] -> w1107
          tunnel: w1106 -> [w1127]
          tunnel: [w1126] -> w1100
          tunnel: w1099 -> [w1126]
          tunnel: [w1125] -> w1092
          tunnel: w1091 -> [w1125]
          tunnel: [w1131] -> w1108
          tunnel: w1107 -> [w1131]
          tunnel: [w1130] -> w1101
          tunnel: w1100 -> [w1130]
          tunnel: [w1129] -> w1093
          tunnel: w1092 -> [w1129]
          tunnel: [w1135] -> w1109
          tunnel: w1108 -> [w1135]
          tunnel: [w1134] -> w1102
          tunnel: w1101 -> [w1134]
          tunnel: [w1133] -> w1094
          tunnel: w1093 -> [w1133]
          tunnel: [w1139] -> w1110
          tunnel: w1109 -> [w1139]
          tunnel: [w1138] -> w1103
          tunnel: w1102 -> [w1138]
          tunnel: [w1137] -> w1095
          tunnel: w1094 -> [w1137]
          tunnel: w1110 -> [w1145]
          tunnel: w1103 -> [w1144]
          tunnel: [w1142] -> w1096
          tunnel: w1095 -> [w1142]
          tunnel: w1096 -> [w1146]
          frame #0 {
            n723 = local read "Laser interlacing mode"() -> (w1113:enum32{"Laser ON", "Laser OFF", "Interlace"})
            n724 = local read "Green FB On/Off"() -> (w1112:bool)
            n725 = local read "Green Laser ON"() -> (w1114:bool)
          }
          frame #1 {
            n726 = property on="Green FB On/Off" class="Bool (strict)"("Val(Sgnl)"=FALSE ("Value (Signaling)")) -> ()  [unwired: 2 in, 2 out]
          }
          frame #2 {
            n727 = property on="Green Laser ON" class="Bool (strict)"("Val(Sgnl)"=TRUE ("Value (Signaling)")) -> ()  [unwired: 2 in, 2 out]
            n728 = property on="Flip Green Filter" class="Bool (strict)"("Val(Sgnl)"=TRUE ("Value (Signaling)")) -> ()  [unwired: 2 in, 2 out]
            n729 = property on="Laser interlacing mode" class="RadioBtnsControl (strict)"("Val(Sgnl)"=enum32{"Laser ON", "Laser OFF", "Interlace"}."Laser ON" ("Value (Signaling)")) -> ()  [unwired: 2 in, 2 out]
          }
          frame #3 {
            n730 = Wait (ms)(milliseconds to wait=u32 500) -> ()  [unwired: 1 out]
          }
          frame #4 {
            n731 = property on="Confocal Image" class="Bool (strict)"("Val(Sgnl)"=TRUE ("Value (Signaling)")) -> ()  [unwired: 2 in, 2 out]
          }
          frame #5 {
            n732 = Wait (ms)(milliseconds to wait=u32 2000) -> ()  [unwired: 1 out]
          }
          frame #6 {
            n733 = while {
              stop <- w1140 stop-if-true
              n734 = local read "Saving..."() -> (w1141:bool)
              n735 = Not(x=w1141) -> (.not. x?=w1140:bool)
            }
          }
          frame #7 {
            n736 = property on="Flip Green Filter" class="Bool (strict)"("Val(Sgnl)"=TRUE ("Value (Signaling)")) -> ()  [unwired: 2 in, 2 out]
            n737 = property on="Green Laser ON" class="Bool (strict)"("Val(Sgnl)"=w1145) -> ()  [unwired: 2 in, 2 out]
            n738 = property on="Laser interlacing mode" class="RadioBtnsControl (strict)"("Val(Sgnl)"=w1144) -> ()  [unwired: 2 in, 2 out]
          }
          frame #8 {
            n739 = property on="Green FB On/Off" class="Bool (strict)"("Val(Sgnl)"=w1146) -> ()  [unwired: 2 in, 2 out]
          }
        }
      }
      event "Move in a Circle": Value Change {
        w1148 = dbl[] []
        # "converting distance (d) to angle (a)\na=arcsin(d/2r)"
        # "radius"
        # "radius"
        # "T1 Y"
        # "T1 X"
        n740 = event-data() -> ()  [unwired: 1 in, 5 out]
        n741 = local read "BD 1 Frequency 1 (MHz)"() -> (w1156:dbl)
        n742 = local read "BD 2 Frequency 1 (MHz)"() -> (w1155:dbl)
        n743 = local read "BD 1 Frequency 2 (MHz)"() -> (w1154:dbl)
        n744 = local read "BD 2 Frequency 2 (MHz)"() -> (w1153:dbl)
        n745 = Subtract(x=w1155, y="Center Y Frequency (MHz)") -> (x-y=w1160:dbl)
        n746 = Absolute Value(x=w1160) -> (abs(x)=w1151:dbl)
        n747 = flat-sequence {
          tunnel: w1151 -> [w1163]
          tunnel: [w1163] -> w1150
          frame #0 {
            n748 = local write "Radius (MHz)"(w1163) -> ()
          }
        }
        n749 = node-c288("Time step (ms)") -> (w1162:T23)  [unwired: 3 in]
        n750 = timed-loop {
          timing: w1162 -> [_]
          timing-out: [_] -> w1161
          tunnel: w1156 -> [w1254]
          tunnel: w1155 -> [_]
          tunnel: w1154 -> [w1258]
          tunnel: w1153 -> [_]
          tunnel: "Center Y Frequency (MHz)" -> [w1247]
          shift-right: [w1208] -> _
          shift-left: w1148 -> [w1215]
          shift-right: [w1206] -> _
          shift-left: w1148 -> [w1214]
          shift-right: [w1199] -> _
          shift-left: w1148 -> [w1212]
          shift-right: [w1197] -> _
          shift-left: w1148 -> [w1211]
          tunnel: "Move in a Circle" -> [_]
          tunnel: ["Back to start on finish?"] -> w1152
          tunnel: w1150 -> [_]
          tunnel: w1149 -> [w1229]
          tunnel: w1148 -> [w1210]
          shift-right: [w1181] -> _
          shift-left: 0.0 -> [w1179]
          i -> [w1188]
          stop <- w1252 stop-if-true
          w1196 = 0 ("index")
          w1217 = 1 ("dimension size")
          # "Keep phase within\n2pi so errors don't \nbuild"
          # "Accumulated\nphase"
          # "Current phase"
          # "Trap 2"
          # "Trap 1"
          # "ignore if N = 0"
          # "r"
          # "r"
          # "r"
          # "r"
          # "\"omega*t\""
          # "Trap 2"
          # "Trap separation (radians)"
          # "Trap 1"
          # "Offset (starts\n at bottom of\n the circle)"
          # "omega"
          n751 = node-c288() -> (w1265:i64)  [unwired: 1 in]
          n752 = Divide(x=w1265, y=1000) -> (x/y=w1184:dbl)
          n753 = Divide(x="2D Motion Trap Separation (MHz)", y="Radius (MHz)") -> (x/y=w1239:dbl)
          n754 = Negate(x=w1184) -> (-x=w1183:dbl)
          n755 = Divide(x="Trap 2 phase shift (deg)", y=360.0) -> (x/y=w1230:dbl)
          n756 = Inverse Sine(1:w1239) -> (0:w1175:dbl)
          n757 = Multiply(x=6.283185307179586, y=w1230) -> (x*y=w1176:dbl)
          n758 = Multiply(x=6.283185307179586, y="2D Motion Frequency (Hz)") -> (x*y=w1187:dbl)
          n759 = Select(t=w1184, s="Counterclockwise/Clockwise", f=w1183) -> (s? t:f=w1186:dbl)
          n760 = Multiply(x=w1187, y=w1186) -> (x*y=w1177:dbl)
          n761 = Select(t=w1175, s="Trap shift\nmethod", f=w1176) -> (s? t:f=w1174:dbl)
          n762 = Add(x=w1177, y=w1179) -> (x+y=w1180:dbl)
          n763 = Add(x=w1180, y=w1174) -> (x+y=w1236:dbl)
          n764 = Add(x=w1180, y=1.5707963267948966) -> (x+y=w1185:dbl)
          n765 = Add(x=w1236, y=1.5707963267948966) -> (x+y=w1249:dbl)
          n766 = Cosine(x=w1185) -> (cos(x)=w1263:dbl)
          n767 = Sine(x=w1185) -> (sin(x)=w1262:dbl)
          n768 = Multiply(x=w1263, y="Radius (MHz)") -> (x*y=w1256:dbl)
          n769 = Cosine(x=w1249) -> (cos(x)=w1261:dbl)
          n770 = Sine(x=w1249) -> (sin(x)=w1260:dbl)
          n771 = Multiply(x=w1262, y="Radius (MHz)") -> (x*y=w1255:dbl)
          n772 = Multiply(x=w1261, y="Radius (MHz)") -> (x*y=w1259:dbl)
          n773 = Multiply(x=w1260, y="Radius (MHz)") -> (x*y=w1257:dbl)
          n774 = Add(x=w1256, y=w1254) -> (x+y=w1205:dbl)
          n775 = Add(x=w1255, y=w1247) -> (x+y=w1203:dbl)
          n776 = Greater Or Equal?(x=w1188, y="N steps then stop") -> (x >= y?=w1246:bool)
          n777 = Add(x=w1259, y=w1258) -> (x+y=w1194:dbl)
          n778 = Add(x=w1257, y=w1247) -> (x+y=w1192:dbl)
          n779 = Not Equal To 0?(x="N steps then stop") -> (x != 0?=w1242:bool)
          n780 = And(x=w1246, y=w1242) -> (x .and. y?=w1243:bool)
          n781 = local read "Trap 1 sum mean"() -> (w1226:dbl)
          n782 = local read "Stop All"() -> (w1251:bool)
          n783 = local write "BD 1 Frequency 1 (MHz)"(w1205) -> ()
          n784 = local write "BD 2 Frequency 1 (MHz)"(w1203) -> ()
          n785 = local write "BD 1 Frequency 2 (MHz)"(w1194) -> ()
          n786 = local write "BD 2 Frequency 2 (MHz)"(w1192) -> ()
          n787 = Select(t=w1188, s="test", f=w1226) -> (s? t:f=→"Waveform Chart":dbl)
          n788 = Compound Arithmetic op=OR(w1251, "Stop Moving", w1243) -> (w1252:bool)
          n789 = local read "BD 1 Frequency 3 (MHz)"() -> (w1235:dbl)
          n790 = local read "BD 2 Frequency 3 (MHz)"() -> (w1234:dbl)
          n791 = Select(t=w1210, s="Reset graph", f=w1211) -> (s? t:f=w1191:dbl[])
          n792 = Select(t=w1210, s="Reset graph", f=w1212) -> (s? t:f=w1193:dbl[])
          n793 = Select(t=w1210, s="Reset graph", f=w1214) -> (s? t:f=w1202:dbl[])
          n794 = Select(t=w1210, s="Reset graph", f=w1215) -> (s? t:f=w1204:dbl[])
          n795 = Initialize Array(w1192, w1217) -> (w1218:dbl[])
          n796 = Initialize Array(w1203, w1217) -> (w1221:dbl[])
          n797 = Initialize Array(w1194, w1217) -> (w1219:dbl[])
          n798 = Initialize Array(w1205, w1217) -> (w1222:dbl[])
          n799 = local read "Y RF Frequency Limits (MHz)"() -> (w1232:T16)
          n800 = local read "X RF Frequency Limits (MHz)"() -> (w1233:T16)
          n801 = call "set RF board frequency - interlace.vi"("Board 2 Frequency Limits"=w1232, "Board 1 Frequency Limits"=w1233, "FPGA VI Reference In"=w1229, "Board 2 Frequency 3 (MHz)"=w1234, "Board 1 Frequency 3 (MHz)"=w1235, "Board 2 Frequency 2 (MHz)"=w1192, "Board 2 Frequency 1 (MHz)"=w1203, "Board 1 Frequency 2 (MHz)"=w1194, "Board 1 Frequency 1  (MHz)"=w1205) -> ()  [unwired: 1 in, 2 out]
          n802 = Bundle(w1219, w1218) -> (w1190:cluster{dbl[], dbl[]})  [unwired: 1 in]
          n803 = Bundle(w1222, w1221) -> (w1220:cluster{dbl[], dbl[]})  [unwired: 1 in]
          n804 = Build Array (concatenate)(w1205, w1204) -> (w1209:dbl[])
          n805 = Build Array (concatenate)(w1203, w1202) -> (w1207:dbl[])
          n806 = Build Array (concatenate)(w1194, w1193) -> (w1200:dbl[])
          n807 = Build Array (concatenate)(w1192, w1191) -> (w1198:dbl[])
          n808 = Bundle(w1209, w1207) -> (w1189:cluster{dbl[], dbl[]})  [unwired: 1 in]
          n809 = Bundle(w1200, w1198) -> (w1216:cluster{dbl[], dbl[]})  [unwired: 1 in]
          n810 = Build Array(w1220, w1190, w1189, w1216) -> (→"Trap trajectories":cluster{dbl[], dbl[]}[])
          n811 = case "To pause the process" shown="True" "Pause rotation" {
            frame False {
            }
            frame True {
              n812 = while {
                stop <- w1268 stop-if-true
                n813 = local read "Pause rotation"() -> (w1269:bool)
                n814 = Wait (ms)(milliseconds to wait=u32 10) -> ()  [unwired: 1 out]
                n815 = Not(x=w1269) -> (.not. x?=w1268:bool)
              }
            }
          }
          n816 = Decrement(x="N steps to plot") -> (x-1=w1195:i32)
          n817 = Array Subset(array=w1207, index=w1196, length=w1195) -> (w1206:dbl[])
          n818 = Array Subset(array=w1209, index=w1196, length=w1195) -> (w1208:dbl[])
          n819 = Array Subset(array=w1200, index=w1196, length=w1195) -> (w1199:dbl[])
          n820 = Array Subset(array=w1198, index=w1196, length=w1195) -> (w1197:dbl[])
          n821 = Quotient & Remainder(x=w1180, y=6.283185307179586) -> (x-y*floor(x/y)=w1181:dbl)  [unwired: 1 out]
          n822 = node-c288() -> ()  [unwired: 1 in, 1 out]
        }
        n823 = node-c288(w1161) -> ()  [unwired: 1 out]
        n824 = case shown="True" w1152 {
          tunnel: w1156 -> [_ w1167]
          tunnel: w1155 -> [_ w1166]
          tunnel: w1154 -> [_ w1165]
          tunnel: w1153 -> [_ w1164]
          frame False {
          }
          frame True {
            n825 = flat-sequence {